vi "UHR-Fleezers Control (host) - 12.0(oscillate_test).vi"() -> ()   [LabVIEW 2014] (continued)
    n3026 = Divide(x=w3808, y=w3807) -> (x/y=→"s/Mean":dbl)
    n3027 = feedback-in #26("Calibration") -> ()
    n3028 = feedback #26(u16 1 ("Calibration")) -> (w3837:u16)
    n3029 = Divide(x="T2 offset_x (mV)", y=1000.0) -> (x/y=w3817:dbl)
    n3030 = case shown="0, Default" "Calibration" {
      tunnel: "T1 a_x (nm/V)" -> [_ w4246 w4267]
      tunnel: "T1 k_x (pN/nm)" -> [_ _ w4257]
      tunnel: "T2 a_x (nm/V)" -> [_ w4245 w4265]
      tunnel: "T2 k_x (pN/nm)" -> [_ _ w4258]
      tunnel: w3818 -> [w4228 w4243 w4263]
      tunnel: w3815 -> [w4227 w4241 w4261]
      tunnel: [w4228 w4240 w4260] -> w3846
      tunnel: [w4227 w4239 w4259] -> w3845
      tunnel: ["T1 X (V)" ("Label.Text") "T1 X (nm)" ("Label.Text") "T1 X (pN)" ("Label.Text")] -> w3834
      tunnel: ["T2 X (V)" ("Label.Text") "T2 X (nm)" ("Label.Text") "T2 X (pN)" ("Label.Text")] -> w3833
      tunnel: ["Position (V)" ("Label.Text") "Position (nm)" ("Label.Text") "Force (pN)" ("Label.Text")] -> w3835
      tunnel: w3817 -> [_ w4231 w4250]
      tunnel: w3819 -> [_ w4234 w4252]
      tunnel: ["Mean (V)" ("Label.Text") "Mean (nm)" ("Label.Text") "Mean (pN)" ("Label.Text")] -> w3830
      tunnel: ["Difference (V)" ("Label.Text") "Difference (nm)" ("Label.Text") "Difference (pN)" ("Label.Text")] -> w3772
      frame 0, Default {
      }
      frame 1 {
        n3031 = Unbundle By Name(w4243) -> ("Y"=w4247:dbl[])
        n3032 = Unbundle By Name(w4241) -> ("Y"=w4232:dbl[])
        n3033 = Subtract(x=w4247, y=w4234) -> (x-y=w4235:dbl[])
        n3034 = Subtract(x=w4232, y=w4231) -> (x-y=w4233:dbl[])
        n3035 = Multiply(x=w4233, y=w4245) -> (x*y=w4242:dbl[])
        n3036 = Multiply(x=w4246, y=w4235) -> (x*y=w4244:dbl[])
        n3037 = Bundle By Name(cluster=w4241, "Y"=w4242) -> (w4239:waveform(dbl))
        n3038 = Bundle By Name(cluster=w4243, "Y"=w4244) -> (w4240:waveform(dbl))
      }
      frame 2 {
        n3039 = Unbundle By Name(w4263) -> ("Y"=w4268:dbl[])
        n3040 = Unbundle By Name(w4261) -> ("Y"=w4266:dbl[])
        n3041 = Subtract(x=w4266, y=w4250) -> (x-y=w4251:dbl[])
        n3042 = Subtract(x=w4268, y=w4252) -> (x-y=w4253:dbl[])
        n3043 = Compound Arithmetic op=MULTIPLY(w4251, w4265, w4258) -> (w4262:dbl[])
        n3044 = Compound Arithmetic op=MULTIPLY(w4257, w4267, w4253) -> (w4264:dbl[])
        n3045 = Bundle By Name(cluster=w4261, "Y"=w4262) -> (w4259:waveform(dbl))
        n3046 = Bundle By Name(cluster=w4263, "Y"=w4264) -> (w4260:waveform(dbl))
      }
    }
    n3047 = Not Equal?(x=w3837, y="Calibration") -> (x != y?=w3798:bool)
    n3048 = case shown="True" w3798 {
      tunnel: w3835 -> [_ w4221]
      tunnel: w3834 -> [_ w4220]
      tunnel: w3833 -> [_ w4219]
      tunnel: w3830 -> [_ w4218]
      tunnel: w3772 -> [_ w4217]
      frame False {
      }
      frame True {
        n3049 = property on="Force" class="WFChart (strict)"("YScale.NameLbl.Text"=w4221) -> ()  [unwired: 2 in, 2 out]
        n3050 = property on="T2 X" class="DigNum (strict)"("Caption.Text"=w4219) -> ()  [unwired: 2 in, 2 out]
        n3051 = property on="T1 X" class="DigNum (strict)"("Caption.Text"=w4220) -> ()  [unwired: 2 in, 2 out]
        n3052 = property on="Mean" class="DigNum (strict)"("Caption.Text"=w4218) -> ()  [unwired: 2 in, 2 out]
        n3053 = property on="Difference" class="DigNum (strict)"("Caption.Text"=w4217) -> ()  [unwired: 2 in, 2 out]
      }
    }
    n3054 = Unbundle By Name(w3818) -> ("Y"=w3821:dbl[])
    n3055 = Unbundle By Name(w3815) -> ("Y"=w3824:dbl[])
    n3056 = Subtract(x=w3821, y=w3819) -> (x-y=w3822:dbl[])
    n3057 = Subtract(x=w3824, y=w3817) -> (x-y=w3823:dbl[])
    n3058 = Multiply(x=w3823, y="T2 a_x (nm/V)") -> (x*y=w3625:dbl[])
    n3059 = Multiply(x="T1 a_x (nm/V)", y=w3822) -> (x*y=w3626:dbl[])
    n3060 = Not(x="Trap Trig. Fl.") -> (.not. x?=w3662:bool)
    n3061 = Multiply(x=w3845, y=-1.0) -> (x*y=w3826:waveform(dbl))
    n3062 = Subtract(x=w3626, y=w3625) -> (x-y=w3814:dbl[])
    n3063 = Unbundle By Name(w3845) -> ("Y"=w3788:dbl[])
    n3064 = Unbundle By Name(w3846) -> ("Y"=w3627:dbl[])
    n3065 = Negate(x=w3814) -> (-x=w3623:dbl[])
    n3066 = Build Array(w3846, w3826) -> (→"Force":waveform(dbl)[])
    n3067 = Subtract(x=w3623, y="Offset (nm)") -> (x-y=w3786:dbl[])
    n3068 = case shown="True" "Read Lateness and Rel Phase" {
      tunnel: w3643 -> [w4192 w4216]
      tunnel: w3642 -> [w4193 w4215]
      tunnel: [w4192 w4214] -> w3812
      tunnel: [w4193 w4213] -> w3811
      frame False {
      }
      frame True {
        n3069 = xnode "Read/Write Control"("FPGA VI Reference In"=w4216, "error in"=w4215) -> ("FPGA VI Reference Out"=w4214:T22, "error out"=w4213:errorcluster, "GI Relative phase"=→"GI relative phase":i16, "Relative phase"=→"Relative phase (AI1)":i16, "AI Late Counter"=→"Late Counter (AI1)":u8, "GI Late Counter"=→"GI Late Counter":u8, "MCL Late Counter"=→"MCL Late Counter":u8, "MCL Relative Phase"=→"Relative Phase (MCL)":i16, "APD Acq Relative Phase"=→"APD Acq Relative Phase":i16, "APD 1 Gate Relative Phase"=→"APD 1 Gate Relative Phase":i16, "APD 2 Gate Relative Phase"=→"APD 2 Gate Relative Phase":i16, "APD Acq Late Counter"=→"APD Acq Late Counter":u8, "APD 1 Gate Late Counter"=→"APD 1 Gate Late Counter":u8, "APD 2 Gate Late Counter"=→"APD 2 Gate Late Counter":u8, "Green FB Relative Phase"=→"Relative phase (Green FB)":i16, "GI Relative phase 2"=→"GI relative phase 2":i16, "GI Late Counter 2"=→"GI Late Counter 2":u8, "Trap Pos FIFO Timeout"=→"Trap Pos FIFO Timeout":u16, "Trap AI FIFO Timeout"=→"Trap AI FIFO Timeout":u16, "RI relative phase"=→"RI relative phase":i16, "RI late counter"=→"RI late counter":u8)
      }
    }
    n3070 = call-poly <vilib>:"Mean.vi"("X"=w3788) -> ("mean"=w3629:dbl)  [unwired: 1 out]
    "T2 X" <- w3629
    n3071 = Negate(x=w3788) -> (-x=w3789:dbl[])
    n3072 = call-poly <vilib>:"Mean.vi"("X"=w3627) -> ("mean"=w3630:dbl)  [unwired: 1 out]
    "T1 X" <- w3630
    n3073 = Negate(x=w3629) -> (-x=w3628:dbl)
    n3074 = Bundle By Name(cluster=w3818, "Y"=w3786) -> (w3763:waveform(dbl))
    "Bead Separation" <- w3763
    n3075 = Add(x=w3627, y=w3789) -> (x+y=w3790:dbl[])
    n3076 = Add(x=w3630, y=w3628) -> (x+y=w3832:dbl)
    n3077 = Subtract(x=w3630, y=w3628) -> (x-y=→"Difference":dbl)
    n3078 = Divide(x=w3790, y=2.0) -> (x/y=→"Vec Mean of T1 T2":dbl[])
    n3079 = Divide(x=w3832, y=2.0) -> (x/y=w3792:dbl)
    "Mean" <- w3792
    n3080 = feedback-in #27("Trap Trig. Fl.") -> ()
    n3081 = feedback #27("Trap Trig. Fl.") -> (w3660:bool)
    n3082 = And(x=w3662, y=w3660) -> (x .and. y?=w3661:bool)
    n3083 = case "If have just turned off triggering" shown="True" w3661 {
      tunnel: w3643 -> [_ w4022]
      tunnel: w3642 -> [_ w4021]
      frame False {
      }
      frame True {
        w4020 = FALSE ("FPGA Trap Trig")
        n3084 = xnode "Read/Write Control"("FPGA VI Reference In"=w4022, "error in"=w4021, "FPGA Trap Trig"=w4020) -> ("FPGA VI Reference Out"=w4019:T22, "error out"=w4018:errorcluster)
        n3085 = xnode "Read/Write Control"("FPGA VI Reference In"=w4019, "error in"=w4018, "TTrig?"=w4020) -> ()  [unwired: 2 out]
        n3086 = local write "Initializing"(FALSE ("Initializing")) -> ()
        n3087 = local write "Triggered"(FALSE ("Triggered")) -> ()
        n3088 = local write "Waiting"(FALSE ("Waiting")) -> ()
      }
    }
    n3089 = Not(x=w3660) -> (.not. x?=w3673:bool)
    n3090 = And(x="Trap Trig. Fl.", y=w3673) -> (x .and. y?=w3670:bool)
    n3091 = local read "Tether"() -> (w3793:bool)
    n3092 = Or(x=w3670, y="Reinitialize") -> (x .or. y?=w3656:bool)
    n3093 = feedback #28(w3666) -> (w3671:string)
    n3094 = Select(t=w3666, s=w3670, f=w3671) -> (s? t:f=w3665:string)
    n3095 = Select(t=w3666, s="Reinitialize", f=w3665) -> (s? t:f=w3664:string)
    n3096 = feedback #29(0) -> (w3668:i32)
    n3097 = feedback #30(w3786) -> (w3785:dbl[])
    n3098 = Build Array (concatenate)(w3786, w3785) -> (w3624:dbl[])
    n3099 = case "For determining if there is a tether still" shown="True" w3793 {
      tunnel: w3792 -> [_ w4146]
      frame False {
      }
      frame True {
        n3100 = Greater?(x="Lost Tether Alarm Threshold (pN)", y=w4146) -> (0:w4144:bool)
        n3101 = case shown="True" w4144 {
          frame False {
          }
          frame True {
            w4147 = TRUE
            w4151 = FALSE ("Multiple tether")
            w4152 = FALSE ("Value (Signaling)")
            n3102 = flat-sequence {
              frame #0 {
                # "stop only if saving"
                n3103 = local read "Saving..."() -> (w4164:bool)
                n3104 = And(x=w4164, y="TA Cancel Save?") -> (x .and. y?=w4163:bool)
                n3105 = local write "Stop Saving"(w4163) -> ()
              }
              frame #1 {
                n3106 = case shown="True" "TA Green Off?" {
                  frame False {
                  }
                  frame True {
                    w4167 = FALSE ("Fl. Triggered...")
                    n3107 = local write "Fl. Triggered..."(w4167) -> ()
                    n3108 = property on="Green ON/Interlacing" class="Bool (strict)"("Val(Sgnl)"=w4167) -> ()  [unwired: 2 in, 2 out]
                  }
                }
              }
            }
            n3109 = local read "Time tether formed"() -> (w4158:timestamp)
            n3110 = Get Date/Time In Seconds() -> (seconds since 1Jan1904=w4159:timestamp)
            n3111 = Subtract(x=w4159, y=w4158) -> (x-y=w4157:dbl)
            n3112 = Number To Decimal String(number=w4157) -> (decimal integer string=w4154:string)  [unwired: 1 out]
            n3113 = local read "Messages"() -> (w4161:string)
            n3114 = call <vilib>:"Beep.vi"("use system alert? (T)"=FALSE, "duration (msec)"=u32 200, "frequency (Hz)"=u32 200) -> ()  [unwired: 9 out]
            n3115 = Concatenate Strings("Lost tether (" ("Message to add"), w4154, " s)." ("string")) -> (w4156:string)
            n3116 = local write "Tether"(FALSE ("Tether")) -> ()
            n3117 = call "Update messages.vi"("Message to add"=w4156, "Old message string"=w4161) -> ("New message string"=w4160:string)
            n3118 = local write "Messages"(w4160) -> ()
            n3119 = local write "Pause dwell"(w4152) -> ()
            n3120 = property on="Fl. Triggered..." class="Bool (strict)"("Val(Sgnl)"=w4152) -> ()  [unwired: 2 in, 2 out]
            n3121 = local write "Dip for Protein"(w4152) -> ()
            n3122 = property on="Trap Pos. FB ON" class="Bool (strict)"("Val(Sgnl)"=w4152) -> ()  [unwired: 2 in, 2 out]
            n3123 = property on="Trap Trig. Fl." class="Bool (strict)"("Val(Sgnl)"=w4152) -> ()  [unwired: 2 in, 2 out]
            n3124 = local write "Multiple tether"(w4151) -> ()
            n3125 = local write "Bad fit"(w4151) -> ()
            n3126 = local write "Hysteresis"(w4151) -> ()
            n3127 = local write "Good tether"(w4151) -> ()
            n3128 = local write "Save scans"(w4147) -> ()
            n3129 = local write "Restart DMA? (AOD)"(w4147) -> ()
          }
        }
      }
    }
    n3130 = case "For triggering actions based on the trap position (e.g., turning the excitation laser on if trap under feedback moves so far)" shown="True" "Trap Trig. Fl." {
      tunnel: w3651 -> [_ w4035]
      tunnel: w3664 -> [_ w4034]
      tunnel: ["" ("t") w4033] -> w3672
      tunnel: w3656 -> [_ w4032]
      tunnel: [0 ("t") w4031] -> w3669
      tunnel: w3668 -> [_ w4030]
      tunnel: w3643 -> [_ w4029]
      tunnel: w3642 -> [_ w4028]
      frame False {
      }
      frame True {
        n3131 = case shown="\"Wait for trigger\"" w4034 {
          tunnel: w4035 -> [w4052 _ _ w4100]
          tunnel: [w4049 w4081 "" ("t") w4103] -> w4033
          tunnel: w4032 -> [_ _ _ w4091]
          tunnel: [w4048 w4078 0 ("t") w4092] -> w4031
          tunnel: w4030 -> [_ w4080 _ w4098]
          tunnel: w4029 -> [w4037 w4075 _ w4094]
          tunnel: w4028 -> [w4036 w4074 _ w4093]
          frame "Wait for trigger" {
            n3132 = local read "Trap Trig. (FPGA)"() -> (w4040:bool)
            n3133 = Subtract(x=w4052, y="Mean T1 Position\nto compare (nm)") -> (x-y=w4045:dbl[])
            n3134 = call <vilib>:"Std Deviation and Variance.vi"("X"=w4045) -> ("mean"=→"mean":dbl, "standard deviation"=→"standard\ndeviation":dbl)  [unwired: 1 in, 1 out]
            n3135 = Array Max & Min(array=w4045) -> (max value=→"max value":dbl, min value=→"min value":dbl)  [unwired: 2 out]
            n3136 = Greater?(x=w4045, y="Threshold (nm)") -> (0:w4055:bool[])
            n3137 = case shown="True" w4040 {
              tunnel: w4037 -> [_ w4061]
              tunnel: w4036 -> [_ w4060]
              tunnel: [FALSE ("TTrig?") w4059] -> w4043
              frame False {
              }
              frame True {
                n3138 = xnode "Read/Write Control"("FPGA VI Reference In"=w4061, "error in"=w4060) -> ("TTrig?"=w4059:bool)  [unwired: 2 out]
              }
            }
            n3139 = Or Array Elements(Boolean array=w4055) -> (logical OR=w4042:bool)
            n3140 = Select(t=w4043, s=w4040, f=w4042) -> (s? t:f=w4041:bool)
            n3141 = Not(x=w4040) -> (.not. x?=w4039:bool)
            n3142 = And(x=w4041, y=w4039) -> (x .and. y?=w4038:bool)
            n3143 = Select(t="Triggered", s=w4041, f="Wait for trigger") -> (s? t:f=w4049:string)
            n3144 = case shown="True" w4041 {
              tunnel: [0 0] -> w4048
              tunnel: w4037 -> [_ w4066]
              tunnel: w4036 -> [_ w4065]
              frame False {
                "Waiting" <- TRUE ("Waiting")
              }
              frame True {
                n3145 = xnode "Read/Write Control"("FPGA VI Reference In"=w4066, "error in"=w4065, "TTrig?"=FALSE) -> ()  [unwired: 2 out]
                n3146 = local read "Messages"() -> (w4069:string)
                n3147 = call <vilib>:"Beep.vi"() -> ()  [unwired: 12 in]
                n3148 = call "Update messages.vi"("Message to add"="Unwinding trigger.", "Old message string"=w4069) -> ("New message string"=w4070:string)
                n3149 = local write "Messages"(w4070) -> ()
                n3150 = local write "Waiting"(FALSE ("Waiting")) -> ()
                "Triggered" <- TRUE ("Triggered")
              }
            }
            n3151 = case "Only need to turn on laser if host triggered" shown="True" w4038 {
              frame False {
              }
              frame True {
                n3152 = property on="Green ON/Interlacing" class="Bool (strict)"("Val(Sgnl)"=TRUE ("Value (Signaling)")) -> ()  [unwired: 2 in, 2 out]
              }
            }
          }
          frame "Triggered" {
            n3153 = local read "Trap Trig. (FPGA)"() -> (w4077:bool)
            n3154 = Increment(x=w4080) -> (x+1=w4078:i32)
            n3155 = Greater Or Equal?(x=w4078, y="Fl. ON time (n)") -> (x >= y?=w4076:bool)
            n3156 = Select(t="Wait for trigger", s=w4076, f="Triggered" ("t")) -> (s? t:f=w4081:string)
            n3157 = And(x=w4076, y=w4077) -> (x .and. y?=w4073:bool)
            n3158 = case shown="True" w4073 {
              tunnel: w4075 -> [_ w4085]
              tunnel: w4074 -> [_ w4084]
              frame False {
              }
              frame True {
                n3159 = xnode "Read/Write Control"("FPGA VI Reference In"=w4085, "error in"=w4084, "FPGA Trap Trig"=TRUE) -> ()  [unwired: 2 out]
              }
            }
            n3160 = case shown="True" w4076 {
              frame False {
              }
              frame True {
                w4087 = FALSE ("Value (Signaling)")
                n3161 = local write "Triggered"(w4087) -> ()
                n3162 = local write "Waiting"(TRUE ("Waiting")) -> ()
                n3163 = property on="Green ON/Interlacing" class="Bool (strict)"("Val(Sgnl)"=w4087) -> ()  [unwired: 2 in, 2 out]
              }
            }
          }
          frame "Do nothing" {
          }
          frame "Initialize", Default {
            n3164 = Increment(x=w4098) -> (x+1=w4102:i32)
            n3165 = Select(t=1, s=w4091, f=w4102) -> (s? t:f=w4092:i32)
            n3166 = feedback #31(w4100) -> (w4106:dbl[])
            n3167 = Build Array (concatenate)(w4100, w4106) -> (w4099:dbl[])
            n3168 = Greater Or Equal?(x=w4092, y="Wait to get offset (n)") -> (x >= y?=w4095:bool)
            n3169 = Select(t=w4100, s=w4091, f=w4099) -> (s? t:f=w4101:dbl[])
            n3170 = feedback-in #31(w4101) -> ()
            n3171 = call-poly <vilib>:"Mean.vi"("X"=w4101) -> ("mean"=w4096:dbl)  [unwired: 1 out]
            n3172 = local write "Mean T1 Position\nto compare (nm)"(w4096) -> ()
            n3173 = case shown="True" w4091 {
              tunnel: w4094 -> [_ w4112]
              tunnel: w4093 -> [_ w4111]
              frame False {
              }
              frame True {
                w4108 = FALSE ("FPGA Trap Trig")
                n3174 = xnode "Read/Write Control"("FPGA VI Reference In"=w4112, "error in"=w4111, "FPGA Trap Trig"=w4108) -> ("FPGA VI Reference Out"=w4110:T22, "error out"=w4109:errorcluster)
                n3175 = xnode "Read/Write Control"("FPGA VI Reference In"=w4110, "error in"=w4109, "TTrig?"=w4108) -> ()  [unwired: 2 out]
              }
            }
            n3176 = Select(t="Wait for trigger", s=w4095, f="Initialize") -> (s? t:f=w4103:string)
            n3177 = case shown="True" w4095 {
              tunnel: w4096 -> [_ w4115]
              tunnel: w4094 -> [_ w4124]
              tunnel: w4093 -> [_ w4123]
              frame False {
                n3178 = local write "Waiting"(FALSE ("Waiting")) -> ()
                "Initializing" <- TRUE ("Initializing")
              }
              frame True {
                n3179 = local read "Threshold (nm)"() -> (w4127:dbl)
                n3180 = local read "AOM X Cal (nm/MHz)"() -> (w4126:dbl)
                n3181 = Add(x=w4115, y=w4127) -> (x+y=w4128:dbl)
                n3182 = Divide(x=w4128, y=w4126) -> (x/y=w4125:dbl)
                n3183 = call "IR AOM freq to word.vi"("Frequency In (MHz)"=w4125) -> ("Frequency Word Out (double)"=w4122:dbl)
                n3184 = local write "Initializing"(FALSE ("Initializing")) -> ()
                n3185 = local write "Waiting"(TRUE ("Waiting")) -> ()
                n3186 = To Quad Integer(1:w4122) -> (0:w4121:i64)
                n3187 = xnode "Read/Write Control"("FPGA VI Reference In"=w4124, "error in"=w4123, "FPGA TTrig Thresh"=w4121) -> ("FPGA VI Reference Out"=w4118:T22, "error out"=w4117:errorcluster)
                n3188 = xnode "Read/Write Control"("FPGA VI Reference In"=w4118, "error in"=w4117, "FPGA Trap Trig"=TRUE) -> ()  [unwired: 2 out]
              }
            }
          }
        }
      }
    }
    n3189 = feedback-in #28(w3672) -> ()
    n3190 = feedback-in #29(w3669) -> ()
    n3191 = Split 1D Array(array=w3624, index=w3686) -> (first subarray=w3782:dbl[])  [unwired: 1 out]
    n3192 = feedback-in #30(w3782) -> ()
    n3193 = call-poly <vilib>:"Mean.vi"("X"=w3782) -> ("mean"=w3781:dbl)  [unwired: 1 out]
    "Bead Mean (nm)" <- w3781
    n3194 = Subtract(x=w3782, y=w3781) -> (x-y=w3780:dbl[])
    n3195 = Square(x=w3780) -> (x^2=w3779:dbl[])
    n3196 = call-poly <vilib>:"Mean.vi"("X"=w3779) -> ("mean"=w3778:dbl)  [unwired: 1 out]
    n3197 = Square Root(x=w3778) -> (sqrt(x)=w3777:dbl)
    n3198 = Multiply(x=10.0, y=w3777) -> (x*y=→"RMS (Å)":dbl)
    n3199 = xnode ("Read/Write Control")("FPGA VI Reference In"=w3812, "error in"=w3811) -> ("FPGA VI Reference Out"=w3654:T22, "error out"=w3653:errorcluster, "AI2 Y Sum Set 1"=w3907:i16, "AI2 Y Sum Set 2"=w3906:i16, "AI1 X Set 1"=w3714:fxp<+/-,16,1>, "AI1 X Set 2"=w3713:fxp<+/-,16,1>, "Trap Pos FB Int Signal"=→"Trap Pos FB Int Signal":fxp<+/-,24,9>, "Trap Pos FB Int-Norm Signal"=→"Trap Pos FB Int-Norm Signal":fxp<+/-,16,1>, "Trap Pos FB Action"=w3707:i64, "Scanning"=→"AOD Scanning":bool, "Scan I"=→"AOD Scan I":u64, "Scanning MCL"=w3909:bool, "Scan I (MCL)"=→"MCL Scan I":u64, "Green FB Sum"=w3849:i16, "Trap Pos FB Action"=w3641:i64, "Wiggling 1"=→"Wiggling T1":bool, "TTrig Fin Thresh"=w3637:i64, "Wiggling 2"=→"Wiggling T2":bool, "Red FB Sum"=w3604:i16)  [unwired: 2 out]
    "MCL Scanning" <- w3909
    "Trap Pos FB Action" <- w3707
    n3200 = local read "FB Trig Integrate"() -> (w3635:u32)
    n3201 = Divide(x=w3849, y=3276.7) -> (x/y=w3603:dbl)
    "Green laser intensity (V)" <- w3603
    n3202 = Divide(x=w3604, y=3276.7) -> (x/y=w3602:dbl)
    "Red laser intensity (V)" <- w3602
    n3203 = Divide(x=w3641, y=w3635) -> (x/y=w3634:dbl)
    "TTrig Sig (Int)" <- w3634
    n3204 = Divide(x=w3637, y=w3635) -> (x/y=w3632:dbl)
    "TTrig Fin Thresh (Int)" <- w3632
    n3205 = local read "AOM X Cal (nm/MHz)"() -> (w3640:dbl)
    n3206 = local read "AI2 (V)"() -> (w3908:cluster{"Set 1":dbl, "Set 2":dbl})
    n3207 = Bundle By Name(cluster=w3908, "Set 1"=w3907, "Set 2"=w3906) -> (w3904:cluster{"Set 1":dbl, "Set 2":dbl})
    n3208 = Divide(x=w3707, y=327.67) -> (x/y=w3619:dbl)
    n3209 = local read "Trap X (AI1)"() -> (w3727:T10)
    n3210 = Bundle(w3603, w3602) -> (→"Excitation laser intensities plot":cluster{dbl, dbl})  [unwired: 1 in]
    n3211 = call "IR AOM word double to freq.vi"("Frequency Word In (double)"=w3632) -> ("Frequency Out (MHz)"=w3631:dbl)
    n3212 = call "IR AOM word double to freq.vi"("Frequency Word In (double)"=w3634) -> ("Frequency Out (MHz)"=w3633:dbl)
    n3213 = Divide(x=w3904, y=3276.7) -> (x/y=w3903:cluster{"Set 1":dbl, "Set 2":dbl})
    n3214 = Multiply(x=w3633, y=w3640) -> (x*y=w3639:dbl)
    "TTrig Sig (nm)" <- w3639
    n3215 = Multiply(x=w3631, y=w3640) -> (x*y=w3638:dbl)
    "TTrig Fin Thresh (nm)" <- w3638
    n3216 = local write "AI2 (V)"(w3903) -> ()
    n3217 = local read "Trap Pos. FB Range"() -> (w3618:T12)
    n3218 = Bundle(cluster=w3727, "Trap 1"=w3714, "Trap 2"=w3713) -> (→"Trap X (AI1)":T10)
    n3219 = Bundle(w3639, w3638) -> (→"TTrig":cluster{dbl, dbl})  [unwired: 1 in]
    n3220 = Unbundle(w3618) -> ("output high"=w3617:fxp<+/-,64,32>)  [unwired: 1 out]
    n3221 = Divide(x=w3619, y=w3617) -> (x/y=→"Action (%)":dbl)
    n3222 = flat-sequence "To save data" {
      tunnel: [w4988] -> w3926
      tunnel: [w4989] -> w3925
      tunnel: w3879 -> [w4961]
      tunnel: w3659 -> [w4986]
      tunnel: ["Save Calibration"] -> w3900
      tunnel: w3897 -> [w4985]
      tunnel: [w4979] -> w3896
      tunnel: [w4976] -> w3895
      tunnel: [w4973] -> w3894
      tunnel: w3878 -> [w4975]
      tunnel: w3796 -> [w4969]
      tunnel: [w4969] -> w3795
      tunnel: ["Start Saving"] -> w3765
      tunnel: [w4963] -> w3699
      tunnel: [w4962] -> w3698
      tunnel: w3926 -> [w5228]
      tunnel: w3925 -> [w5227]
      tunnel: w3700 -> [w5226]
      tunnel: w3900 -> [w5225]
      tunnel: w3896 -> [w5223]
      tunnel: w3895 -> [w5222]
      tunnel: w3894 -> [w5221]
      tunnel: w3774 -> [w5220]
      tunnel: w3805 -> [w5219]
      tunnel: w3795 -> [w5218]
      tunnel: w3765 -> [w5217]
      tunnel: w3763 -> [w5216]
      tunnel: w3741 -> [w5215]
      tunnel: w3699 -> [w5214]
      tunnel: w3698 -> [w5213]
      tunnel: w3697 -> [w5212]
      tunnel: w3620 -> [w5211]
      frame #0 {
        n3223 = Or(x="Save N Sets", y="Start Saving") -> (x .or. y?=w4970:bool)
        n3224 = To Double Precision Float(number=w4985) -> (double precision float=w4980:dbl)
        n3225 = Build Array(w4970, "Save Calibration", w4961, w4975) -> (w4984:bool[])
        n3226 = Compound Arithmetic op=OR("Save Calibration", w4961, w4970, w4975) -> (w4987:bool)
        n3227 = Boolean Array To Number(Boolean array=w4984) -> (number=w4982:u32)
        n3228 = feedback #32(FALSE ("Save APD Data\nwith Trap Data")) -> (w4964:bool)
        n3229 = feedback #33(refnum<k0> refnum) -> (w4990:refnum<file>)
        n3230 = feedback #34(refnum<k0> refnum) -> (w4966:refnum<file>)
        n3231 = feedback #35(FALSE ("Save APD Data\nwith Trap Data")) -> (w4974:bool)
        n3232 = feedback #36(refnum<k0> refnum) -> (w4977:refnum<file>)
        n3233 = feedback #37(0) -> (w4992:i32)
        n3234 = feedback #38() -> (w4981:u32)  [unwired: 1 out]
        n3235 = case shown="True" w4987 {
          tunnel: [w4999 1] -> w4988
          tunnel: w4992 -> [w5001 _]
          tunnel: [w5000 w5019] -> w4989
          tunnel: w4990 -> [w5000 _]
          tunnel: w4986 -> [_ w5039]
          tunnel: w4980 -> [_ w5037]
          tunnel: w4982 -> [_ w5040]
          tunnel: [w4998 w5018] -> w4979
          tunnel: w4981 -> [w4998 _]
          tunnel: [w4997 w5016] -> w4976
          tunnel: w4977 -> [w4997 _]
          tunnel: [w4996 w5015] -> w4973
          tunnel: w4974 -> [w4996 _]
          tunnel: "Start Saving" -> [_ w5013]
          tunnel: w4969 -> [_ w5012]
          tunnel: [w4995 w5003] -> w4962
          tunnel: w4966 -> [w4995 _]
          tunnel: [w4994 w5002] -> w4963
          tunnel: w4964 -> [w4994 _]
          frame False {
            n3236 = Increment(x=w5001) -> (x+1=w4999:i32)
          }
          frame True {
            w5009 = FALSE ("Start Saving")
            w5014 = 9.0  # File Version
            w5022 = FALSE ("prepend array or string size? (T)")
            w5020 = T29."big-endian, network order" ("byte order (0:big-endian, network order)")
            n3237 = local read "BD 1 Frequency 1 (MHz)"() -> (w5036:dbl)
            n3238 = local read "BD 2 Frequency 1 (MHz)"() -> (w5035:dbl)
            n3239 = local read "BD 1 Frequency 2 (MHz)"() -> (w5034:dbl)
            n3240 = local read "BD 2 Frequency 2 (MHz)"() -> (w5033:dbl)
            n3241 = local read "BD 1 Frequency 3 (MHz)"() -> (w5032:dbl)
            n3242 = local read "BD 2 Frequency 3 (MHz)"() -> (w5031:dbl)
            n3243 = Array Size(array=w5012) -> (size(s)=w5011:i32)
            n3244 = To Double Precision Float(number=w5011) -> (double precision float=w5010:dbl)
            n3245 = local write "Save Calibration"(w5009) -> ()
            n3246 = local write "Start Saving"(w5009) -> ()
            n3247 = Build Array("Save APD Data\nwith Trap Data", "Save Trap Pos. Data") -> (w5006:bool[])
            n3248 = Boolean Array To Number(Boolean array=w5006) -> (number=w5005:u32)
            n3249 = Build Array(w5036, w5035, w5034, w5033, w5032, w5031) -> (w5030:dbl[])
            n3250 = case shown="1, Default" w5040 {
              tunnel: w5039 -> [w5113 w5135 w5151 w5189]
              tunnel: w5010 -> [w5118 w5142 w5171 w5208]
              tunnel: w5037 -> [w5117 w5141 w5170 w5207]
              tunnel: [w5114 w5137 w5162 w5199] -> w5028
              tunnel: [w5106 "Cal sets to save" w5152 w5190] -> w5018
              tunnel: w5030 -> [w5115 w5138 w5164 w5201]
              tunnel: "Save APD Data\nwith Trap Data" -> [w5112 _ w5148 w5187]
              tunnel: [w5112 FALSE ("Save APD Data\nwith Trap Data") w5148 w5187] -> w5015
              tunnel: w5014 -> [w5109 w5132 w5146 w5185]
              tunnel: w5013 -> [w5108 _ _ _]
              tunnel: [w5100 "Active cal?" w5145 w5175] -> w5002
              tunnel: "Save Trap Pos. Data" -> [w5100 _ w5145 w5175]
              tunnel: w5005 -> [w5099 _ w5144 w5174]
              frame 1, Default {
                # "timeseries"
                n3251 = case shown="True" "Profile" {
                  tunnel: [w5121 w5125] -> w5104
                  tunnel: [w5121 w5124] -> w5103
                  tunnel: [w5121 w5123] -> w5102
                  tunnel: [w5121 w5122] -> w5101
                  frame False {
                    w5121 = 0.0 ("f")
                  }
                  frame True {
                    n3252 = local read "Current Position"() -> (w5126:cluster{dbl, dbl, dbl})
                    n3253 = local read "Y change (mm)"() -> (w5122:dbl)
                    n3254 = Unbundle(w5126) -> (w5125:dbl, w5124:dbl, w5123:dbl)
                  }
                }
                n3255 = local read "Save ave N"() -> (w5120:dbl)
                n3256 = Multiply(x=w5120, y=w5113) -> (x*y=w5119:dbl)
                n3257 = To Double Precision Float(number=w5099) -> (double precision float=w5111:dbl)
                n3258 = Select(t=4.0, s="Profile", f=0.0) -> (s? t:f=w5095:dbl)
                n3259 = Build Array(w5109, w5113, w5119, w5118, w5117, w5095) -> (w5116:dbl[])
                n3260 = Build Array(w5111, w5104, w5103, w5102, w5101) -> (w5110:dbl[])
                n3261 = Select(t=u32 4000000000, s=w5108, f="N sets to save") -> (s? t:f=w5106:u32)
                n3262 = Build Array (concatenate)(w5116, w5115, w5110) -> (w5114:dbl[])
              }
              frame 2 {
                w5134 = 0.0 ("f")
                # "If doing active calibration,\nalso save trap position file"
                # "calibration"
                n3263 = property on="Wiggle" class="Bool (strict)"("Val(Sgnl)"="Active cal?") -> ()  [unwired: 2 in, 2 out]
                n3264 = Select(t=2.0, s="Active cal?", f=0.0) -> (s? t:f=w5128:dbl)
                n3265 = Build Array(w5128, w5134, w5134, w5134, w5134) -> (w5133:dbl[])
                n3266 = Build Array(w5132, w5135, w5135, w5142, w5141, 1.0 ("t")) -> (w5139:dbl[])
                n3267 = Build Array (concatenate)(w5139, w5138, w5133) -> (w5137:dbl[])
                "Calibrating..." <- TRUE ("Calibrating...")
              }
              frame 4 {
                w5149 = 0.0 ("f")
                # "scan dir (x/y = 0/1)"
                # "cycles/step"
                # "n scans (f/b)"
                # "steps"
                # "freq. range"
                # "AOD raster scan"
                n3268 = local read "Number of F/B Scans (AOD)"() -> (w5156:u16)
                n3269 = local read "Cycles/step (AOD)"() -> (w5158:u64)
                n3270 = local read "Scan Range (MHz)"() -> (w5161:dbl)
                n3271 = local read "Scan steps (AOD)"() -> (w5160:u64)
                n3272 = local read "Scan BD"() -> (w5168:bool)
                n3273 = local read "Save ave N"() -> (w5173:dbl)
                n3274 = Boolean To (0,1)(Boolean=w5168) -> (0, 1=w5167:i16)
                n3275 = To Double Precision Float(number=w5156) -> (double precision float=w5155:dbl)
                n3276 = To Double Precision Float(number=w5160) -> (double precision float=w5159:dbl)
                n3277 = To Double Precision Float(number=w5158) -> (double precision float=w5157:dbl)
                n3278 = To Double Precision Float(number=w5167) -> (double precision float=w5166:dbl)
                n3279 = Multiply(x=w5173, y=w5151) -> (x*y=w5172:dbl)
                n3280 = To Double Precision Float(number=w5144) -> (double precision float=w5150:dbl)
                n3281 = Build Array(w5150, w5149, w5149, w5149, w5149) -> (w5147:dbl[])
                n3282 = local read "N sets should be saved"() -> (w5153:dbl)
                n3283 = Build Array(w5166, w5161, w5159, w5157, w5155) -> (w5163:dbl[])
                n3284 = Build Array(w5146, w5151, w5172, w5171, w5170, 2.0 ("t")) -> (w5165:dbl[])
                n3285 = Round Toward +Infinity(x=w5153) -> (ceil(x): smallest int >= x=w5154:dbl)
                n3286 = Build Array (concatenate)(w5165, w5164, w5147, w5163) -> (w5162:dbl[])
                n3287 = To Unsigned Long Integer(number=w5154) -> (unsigned 32bit integer=w5152:u32)
              }
              frame 8 {
                w5182 = 0.0 ("f")
                # "MCL raster scan"
                n3288 = local read "Number of scans (MCL)"() -> (w5177:u64)
                n3289 = local read "Scan lines (y)"() -> (w5176:u64)
                n3290 = local read "2D or 1D Scan"() -> (w5179:bool)
                n3291 = local read "Scan Range (V)\n(of steps)"() -> (w5198:dbl)
                n3292 = local read "Fast Scan Dir"() -> (w5205:bool)
                n3293 = local read "Cycles/step (MCL)"() -> (w5195:u64)
                n3294 = local read "Scan steps (MCL)"() -> (w5197:u64)
                n3295 = Select(t=w5176, s=w5179, f=w5177) -> (s? t:f=w5178:u64)
                n3296 = Boolean To (0,1)(Boolean=w5179) -> (0, 1=w5181:i16)
                n3297 = local read "Save ave N"() -> (w5210:dbl)
                n3298 = local read "Initial X"() -> (w5184:dbl)
                n3299 = local read "Initial Y"() -> (w5183:dbl)
                n3300 = To Double Precision Float(number=w5181) -> (double precision float=w5180:dbl)
                n3301 = Boolean To (0,1)(Boolean=w5205) -> (0, 1=w5204:i16)
                n3302 = To Double Precision Float(number=w5178) -> (double precision float=w5193:dbl)
                n3303 = To Double Precision Float(number=w5197) -> (double precision float=w5196:dbl)
                n3304 = To Double Precision Float(number=w5195) -> (double precision float=w5194:dbl)
                n3305 = To Double Precision Float(number=w5204) -> (double precision float=w5203:dbl)
                n3306 = Multiply(x=w5210, y=w5189) -> (x*y=w5209:dbl)
                n3307 = To Double Precision Float(number=w5174) -> (double precision float=w5188:dbl)
                n3308 = local read "N sets should be saved (MCL)"() -> (w5191:dbl)
                n3309 = Build Array(w5188, w5180, w5182, w5182, w5182) -> (w5186:dbl[])
                n3310 = Build Array(w5203, w5198, w5196, w5194, w5193, w5184, w5183) -> (w5200:dbl[])
                n3311 = Build Array(w5185, w5189, w5209, w5208, w5207, 3.0 ("t")) -> (w5202:dbl[])
                n3312 = Round Toward +Infinity(x=w5191) -> (ceil(x): smallest int >= x=w5192:dbl)
                n3313 = Build Array (concatenate)(w5202, w5201, w5186, w5200) -> (w5199:dbl[])
                n3314 = To Unsigned Long Integer(number=w5192) -> (unsigned 32bit integer=w5190:u32)
              }
            }
            n3315 = local read "Index"() -> (w5045:dbl)
            n3316 = call "Create new save file.vi"("Insert"="", "Ext"=".dat", "Index In"=w5045) -> ("Path Out"=w5004:path, "Index Out"=w5017:dbl)
            n3317 = local write "Save file name"(w5004) -> ()
            n3318 = local write "Index"(w5017) -> ()
            n3319 = local write "Save index"(w5017) -> ()
            n3320 = Array Size(array=w5028) -> (size(s)=w5029:i32)
            n3321 = Open/Create/Replace File(file path (use dialog)=w5004, operation (0:open)=T30."create", access (0:read/write)=enum16{"read/write", "read-only", "write-only"}."write-only") -> (refnum out=w5042:refnum<file>)  [unwired: 1 in, 4 out]
            n3322 = local write "Saving..."(TRUE ("Saving...")) -> ()
            n3323 = To Double Precision Float(number=w5029) -> (double precision float=w5027:dbl)
            n3324 = String Length(string="Comment (data description)") -> (length=w5025:i32)
            n3325 = To Double Precision Float(number=w5025) -> (double precision float=w5024:dbl)
            n3326 = Deny Access(7:w5042) -> (3:w5041:refnum<file>)  [unwired: 1 in, 2 out]
            n3327 = Build Array (concatenate)(w5027, w5028, w5024) -> (w5026:dbl[])
            n3328 = case "If fluorescence data to be saved" shown="True" w5015 {
              tunnel: w5004 -> [_ w5094]
              tunnel: [refnum<k0> refnum w5074] -> w5016
              frame False {
              }
              frame True {
                w5073 = 0.0
                n3329 = local read "APD Integration Time (s)"() -> (w5079:dbl)
                n3330 = local read "N APD Samp/step"() -> (w5072:dbl)
                n3331 = Path To String(path=w5094) -> (string=w5093:string)
                n3332 = String Length(string=w5093) -> (length=w5092:i32)
                n3333 = Subtract(x=w5092, y=4) -> (x-y=w5090:i32)
                n3334 = String Subset(string=w5093, length (rest)=w5090) -> (substring=w5089:string)  [unwired: 1 out]
                n3335 = Build Array(w5079, w5072, w5073, w5073, w5073, w5073, w5073, w5073) -> (w5076:dbl[])
                n3336 = Concatenate Strings(w5089, "_fl.dat" ("string")) -> (w5087:string)
                n3337 = Array Size(array=w5076) -> (size(s)=w5078:i32)
                n3338 = String To Path(string=w5087) -> (path=w5083:path)
                n3339 = Open/Create/Replace File(file path (use dialog)=w5083, operation (0:open)=T30."create", access (0:read/write)=enum16{"read/write", "read-only", "write-only"}."write-only") -> (refnum out=w5084:refnum<file>)  [unwired: 1 in, 4 out]
                n3340 = Deny Access(7:w5084) -> (3:w5080:refnum<file>)  [unwired: 1 in, 2 out]
                n3341 = To Double Precision Float(number=w5078) -> (double precision float=w5077:dbl)
                n3342 = Build Array (concatenate)(w5077, w5076) -> (w5075:dbl[])
                n3343 = Write to Binary File(file (use dialog)=w5080, data=w5075, 5:FALSE ("prepend array or string size? (T)"), 9:T29."big-endian, network order" ("byte order (0:big-endian, network order)")) -> (refnum out=w5074:refnum<file>)  [unwired: 1 in, 3 out]
              }
            }
            n3344 = case shown="True" w5002 {
              tunnel: w5004 -> [_ w5056]
              tunnel: [refnum<k0> refnum w5055] -> w5003
              frame False {
              }
              frame True {
                w5051 = 0.0 ("element")
                n3345 = Path To String(path=w5056) -> (string=w5070:string)
                n3346 = Build Array(w5051, w5051, w5051, w5051, w5051, w5051, w5051, w5051) -> (w5052:dbl[])
                n3347 = String Length(string=w5070) -> (length=w5069:i32)
                n3348 = Subtract(x=w5069, y=4) -> (x-y=w5067:i32)
                n3349 = Array Size(array=w5052) -> (size(s)=w5054:i32)
                n3350 = String Subset(string=w5070, length (rest)=w5067) -> (substring=w5066:string)  [unwired: 1 out]
                n3351 = To Double Precision Float(number=w5054) -> (double precision float=w5053:dbl)
                n3352 = Concatenate Strings(w5066, "_pos.dat" ("string")) -> (w5064:string)
                n3353 = Build Array (concatenate)(w5053, w5052) -> (w5050:dbl[])
                n3354 = String To Path(string=w5064) -> (path=w5060:path)
                n3355 = Open/Create/Replace File(file path (use dialog)=w5060, operation (0:open)=T30."create", access (0:read/write)=enum16{"read/write", "read-only", "write-only"}."write-only") -> (refnum out=w5061:refnum<file>)  [unwired: 1 in, 4 out]
                n3356 = Deny Access(7:w5061) -> (3:w5057:refnum<file>)  [unwired: 1 in, 2 out]
                n3357 = Write to Binary File(file (use dialog)=w5057, data=w5050, 5:FALSE ("prepend array or string size? (T)"), 9:T29."big-endian, network order" ("byte order (0:big-endian, network order)")) -> (refnum out=w5055:refnum<file>)  [unwired: 1 in, 3 out]
              }
            }
            n3358 = Write to Binary File(file (use dialog)=w5041, data=w5026, 5:w5022, 9:w5020) -> (refnum out=w5023:refnum<file>)  [unwired: 1 in, 3 out]
            n3359 = Write to Binary File(file (use dialog)=w5023, data="Comment (data description)", 5:w5022, 9:w5020) -> (refnum out=w5019:refnum<file>)  [unwired: 1 in, 3 out]
          }
        }
        n3360 = feedback-in #32(w4963) -> ()
        n3361 = feedback-in #33(w4989) -> ()
        n3362 = feedback-in #34(w4962) -> ()
        n3363 = feedback-in #35(w4973) -> ()
        n3364 = feedback-in #36(w4976) -> ()
        n3365 = feedback-in #37(w4988) -> ()
        n3366 = feedback-in #38(w4979) -> ()
      }
      frame #1 {
        n3367 = local read "Saving..."() -> (w5224:bool)
        n3368 = case shown="True" w5224 {
          tunnel: w5228 -> [_ w5240]
          tunnel: w5227 -> [_ w5253]
          tunnel: w5226 -> [_ w5249]
          tunnel: w5225 -> [_ w5248]
          tunnel: w5223 -> [_ w5229]
          tunnel: w5222 -> [_ w5243]
          tunnel: w5221 -> [_ w5242]
          tunnel: w5220 -> [_ w5241]
          tunnel: w5219 -> [_ w5239]
          tunnel: w5218 -> [_ w5237]
          tunnel: w5217 -> [_ w5236]
          tunnel: w5216 -> [_ w5235]
          tunnel: w5215 -> [_ w5234]
          tunnel: w5214 -> [_ w5233]
          tunnel: w5213 -> [_ w5232]
          tunnel: w5212 -> [_ w5231]
          tunnel: w5211 -> [_ w5230]
          frame False {
          }
          frame True {
            n3369 = Multiply(x=w5240, y=w5239) -> (x*y=→"Time (s)":dbl)
            n3370 = Less Or Equal?(x=w5240, y=w5229) -> (x <= y?=w5251:bool)
            n3371 = Or(x="Stop Saving", y="Abort save 2") -> (x .or. y?=w5244:bool)
            n3372 = Not(x=w5244) -> (.not. x?=w5252:bool)
            n3373 = And(x=w5251, y=w5252) -> (x .and. y?=w5250:bool)
            n3374 = case shown="True" w5250 {
              tunnel: w5253 -> [w5261 w5336]
              tunnel: [0.0 w5339] -> w5247
              tunnel: w5240 -> [_ w5337]
              tunnel: w5229 -> [_ w5338]
              tunnel: w5249 -> [_ w5333]
              tunnel: w5248 -> [_ _]
              tunnel: w5243 -> [w5259 w5326]
              tunnel: w5242 -> [w5258 w5327]
              tunnel: w5241 -> [_ w5325]
              tunnel: w5237 -> [_ w5324]
              tunnel: w5236 -> [_ w5268]
              tunnel: w5235 -> [_ w5317]
              tunnel: w5234 -> [_ w5295]
              tunnel: w5233 -> [w5255 w5277]
              tunnel: w5232 -> [w5256 w5276]
              tunnel: w5231 -> [_ w5273]
              tunnel: w5230 -> [_ w5271]
              frame False {
                w5257 = FALSE
                n3375 = Close File(refnum=w5261) -> ()  [unwired: 1 in, 2 out]
                n3376 = case shown="True" w5258 {
                  tunnel: w5259 -> [_ w5263]
                  frame False {
                  }
                  frame True {
                    n3377 = Close File(refnum=w5263) -> ()  [unwired: 1 in, 2 out]
                  }
                }
                n3378 = case shown="True" w5255 {
                  tunnel: w5256 -> [_ w5262]
                  frame False {
                  }
                  frame True {
                    n3379 = Close File(refnum=w5262) -> ()  [unwired: 1 in, 2 out]
                  }
                }
                n3380 = call <vilib>:"Beep.vi"() -> ()  [unwired: 3 in, 9 out]
                n3381 = local write "Raster Scanning..."(w5257) -> ()
                n3382 = local write "Calibrating..."(w5257) -> ()
                n3383 = property on="Abort wiggle" class="Bool (strict)"("Val(Sgnl)"=TRUE) -> ()  [unwired: 2 in, 2 out]
                n3384 = local write "Stop Saving"(w5257) -> ()
                "Saving..." <- w5257
              }
              frame True {
                n3385 = local read "Calibrating..."() -> (w5328:bool)
                n3386 = case "Write fl. data" shown="True" w5327 {
                  tunnel: w5326 -> [_ w5362]
                  tunnel: w5325 -> [_ w5361]
                  frame False {
                  }
                  frame True {
                    n3387 = Write to Binary File(file (use dialog)=w5362, data=w5361, 5:FALSE ("prepend array or string size? (T)"), 9:T29."big-endian, network order" ("byte order (0:big-endian, network order)")) -> ()  [unwired: 1 in, 4 out]
                  }
                }
                n3388 = Greater?(x="Save ave N", y=1.0) -> (0:w5331:bool)
                n3389 = Not(x=w5328) -> (.not. x?=w5330:bool)
                n3390 = And(x=w5330, y=w5331) -> (x .and. y?=w5274:bool)
                n3391 = case shown="True" w5274 {
                  tunnel: w5273 -> [w5342 w5353]
                  tunnel: [w5342 w5345] -> w5272
                  tunnel: "Save ave N" -> [_ w5346]
                  frame False {
                  }
                  frame True {
                    w5343 = 2 ("dimension size")
                    n3392 = Array Size(array=w5353) -> (size(s)=w5347:i32)
                    n3393 = Divide(x=w5347, y=w5343) -> (x/y=w5351:dbl)
                    n3394 = Reshape Array(w5353, w5351, w5343) -> (w5352:u64[][])
                    n3395 = Transpose 2D Array(2D array=w5352) -> (transposed array=w5350:u64[][])
                    n3396 = for {
                      tunnel: w5350 -> [w5355] mode=indexing
                      tunnel: [w5354] -> w5344 mode=indexing
                      tunnel: w5346 -> [w5356]
                      workers-P: _ -> [_]
                      n3397 = call "downsample 1D array - U64.vi"("Ave N"=w5356, "Array In"=w5355) -> ("Array Out"=w5354:u64[])  [unwired: 1 in]
                    }
                    n3398 = Transpose 2D Array(2D array=w5344) -> (transposed array=w5349:u64[][])
                    n3399 = Divide(x=w5347, y=w5346) -> (x/y=w5348:dbl)
                    n3400 = Reshape Array(w5349, w5348) -> (w5345:u64[])
                  }
                }
                n3401 = case shown="True" w5274 {
                  tunnel: w5333 -> [w5365 w5377]
                  tunnel: [w5365 w5369] -> w5329
                  tunnel: "Save ave N" -> [_ w5370]
                  tunnel: w5324 -> [_ w5368]
                  frame False {
                  }
                  frame True {
                    n3402 = Array Size(array=w5377) -> (size(s)=w5371:i32)
                    n3403 = Array Size(array=w5368) -> (size(s)=w5367:i32)
                    n3404 = Divide(x=w5371, y=w5367) -> (x/y=w5375:dbl)
                    n3405 = Reshape Array(w5377, w5375, w5367) -> (w5376:i16[][])
                    n3406 = Transpose 2D Array(2D array=w5376) -> (transposed array=w5374:i16[][])
                    n3407 = for {
                      tunnel: w5374 -> [w5380] mode=indexing
                      tunnel: [w5379] -> w5366 mode=indexing
                      tunnel: w5370 -> [w5378]
                      workers-P: _ -> [_]
                      n3408 = call "downsample 1D array - I16.vi"("Ave N"=w5378, "Array In"=w5380) -> ("Array Out"=w5379:i16[])  [unwired: 1 out]
                    }
                    n3409 = Transpose 2D Array(2D array=w5366) -> (transposed array=w5373:i16[][])
                    n3410 = Divide(x=w5371, y=w5370) -> (x/y=w5372:dbl)
                    n3411 = Reshape Array(w5373, w5372) -> (w5369:i16[])
                  }
                }
                n3412 = Index Array(array=w5295, index=1) -> (element=w5298:waveform(dbl))
                n3413 = Index Array(array=w5295, index=0) -> (element=w5300:waveform(dbl))
                n3414 = Unbundle By Name(w5298) -> ("Y"=w5302:dbl[])
                n3415 = Unbundle By Name(w5300) -> ("Y"=w5310:dbl[])
                n3416 = case "Write trap pos. data" shown="True" w5277 {
                  tunnel: w5276 -> [_ w5358]
                  tunnel: w5272 -> [_ w5357]
                  frame False {
                  }
                  frame True {
                    n3417 = Write to Binary File(file (use dialog)=w5358, data=w5357, 5:FALSE ("prepend array or string size? (T)"), 9:T29."big-endian, network order" ("byte order (0:big-endian, network order)")) -> ()  [unwired: 1 in, 4 out]
                  }
                }
                n3418 = Write to Binary File(file (use dialog)=w5336, data=w5329, 5:FALSE ("prepend array or string size? (T)"), 9:T29."big-endian, network order" ("byte order (0:big-endian, network order)")) -> ()  [unwired: 1 in, 4 out]
                n3419 = feedback #39(w5302) -> (w5304:dbl[])
                n3420 = Build Array (concatenate)(w5304, w5302) -> (w5303:dbl[])
                n3421 = Select(t=w5302, s=w5268, f=w5303) -> (s? t:f=w5288:dbl[])
                n3422 = feedback-in #39(w5288) -> ()
                n3423 = feedback #40(w5310) -> (w5323:dbl[])
                n3424 = Build Array (concatenate)(w5323, w5310) -> (w5322:dbl[])
                n3425 = Select(t=w5310, s=w5268, f=w5322) -> (s? t:f=w5297:dbl[])
                n3426 = feedback-in #40(w5297) -> ()
                n3427 = Divide(x=w5337, y=w5338) -> (x/y=w5340:dbl)
                n3428 = Multiply(x=w5340, y=100.0) -> (x*y=w5339:dbl)
                n3429 = Build Array(w5297, w5288) -> (→"Saved APD":dbl[][])
                n3430 = Array Size(array=w5297) -> (size(s)=w5315:i32)
                n3431 = Unbundle By Name(w5317) -> ("Y"=w5321:dbl[])
                n3432 = Subtract(x=w5315, y="N pts to average") -> (x-y=w5291:i32)
                n3433 = Multiply(x="N pts to average", y=u16 2) -> (x*y=w5292:u16)
                n3434 = Subtract(x=w5315, y=w5292) -> (x-y=w5290:i32)
                n3435 = feedback #41(w5321) -> (w5320:dbl[])
                n3436 = Build Array (concatenate)(w5320, w5321) -> (w5319:dbl[])
                n3437 = Select(t=w5321, s=w5268, f=w5319) -> (s? t:f=w5318:dbl[])
                "Trap Delta Graph" <- w5318
                n3438 = feedback-in #41(w5318) -> ()
                n3439 = Array Subset(array=w5297, index=w5291, length="N pts to average") -> (w5314:dbl[])
                n3440 = Array Subset(array=w5297, index=w5290, length="N pts to average") -> (w5313:dbl[])
                n3441 = Array Subset(array=w5288, index=w5291, length="N pts to average") -> (w5294:dbl[])
                n3442 = Array Subset(array=w5288, index=w5290, length="N pts to average") -> (w5293:dbl[])
                n3443 = Index Array(array=w5271, index=0) -> (element=w5269:waveform(dbl))
                n3444 = call-poly <vilib>:"Mean.vi"("X"=w5314) -> ("mean"=w5312:dbl)  [unwired: 1 out]
                n3445 = call-poly <vilib>:"Mean.vi"("X"=w5294) -> ("mean"=w5287:dbl)  [unwired: 1 out]
                n3446 = call-poly <vilib>:"Mean.vi"("X"=w5313) -> ("mean"=w5311:dbl)  [unwired: 1 out]
                n3447 = call-poly <vilib>:"Mean.vi"("X"=w5293) -> ("mean"=w5286:dbl)  [unwired: 1 out]
                n3448 = Unbundle By Name(w5269) -> ("Y"=w5266:dbl[])
                n3449 = Subtract(x=w5287, y=w5286) -> (x-y=w5278:dbl)
                "Delta Fl. 2" <- w5278
                n3450 = Subtract(x=w5312, y=w5311) -> (x-y=w5309:dbl)
                "Delta Fl. 1" <- w5309
                n3451 = Initialize Array(w5309, 1 ("dimension size")) -> (w5306:dbl[])
                n3452 = Initialize Array(w5278, 1 ("dimension size")) -> (w5283:dbl[])
                n3453 = feedback #42(w5306) -> (w5307:dbl[])
                n3454 = Build Array (concatenate)(w5307, w5306) -> (w5305:dbl[])
                n3455 = feedback #43(w5283) -> (w5284:dbl[])
                n3456 = Build Array (concatenate)(w5284, w5283) -> (w5282:dbl[])
                n3457 = feedback #44(w5266) -> (w5265:dbl[])
                n3458 = Build Array (concatenate)(w5265, w5266) -> (w5267:dbl[])
                n3459 = Select(t=w5266, s=w5268, f=w5267) -> (s? t:f=w5264:dbl[])
                "Saved trap pos" <- w5264
                n3460 = feedback-in #44(w5264) -> ()
                n3461 = Select(t=w5306, s=w5268, f=w5305) -> (s? t:f=w5281:dbl[])
                n3462 = feedback-in #42(w5281) -> ()
                n3463 = Select(t=w5283, s=w5268, f=w5282) -> (s? t:f=w5280:dbl[])
                n3464 = feedback-in #43(w5280) -> ()
                n3465 = Build Array(w5281, w5280) -> (→"Save APD Deriv":dbl[][])
              }
            }
            "Progress" <- w5247
            "Progress 2" <- w5247
          }
        }
      }
    }
    n3466 = local read "wait to reset values"() -> (w3911:bool)
    n3467 = Not(x=w3909) -> (.not. x?=w3912:bool)
    n3468 = And(x=w3912, y=w3911) -> (x .and. y?=w3913:bool)
    n3469 = case "Part of MCL raster scanning: returns to initial positions after scan done" shown="True" w3913 {
      tunnel: w3654 -> [w4782 w4789]
      tunnel: [w4782 w4788] -> w3915
      tunnel: w3653 -> [w4781 w4787]
      tunnel: [w4781 w4786] -> w3910
      frame False {
      }
      frame True {
        w4797 = 10.0 ("y")
        w4796 = 32767.0 ("y")
        # "to return scan values\nafter a synchronous \nAOM scan"
        n3470 = local read "AO2"() -> (w4790:dbl)
        n3471 = local read "AO1"() -> (w4791:dbl)
        n3472 = local write "wait to reset values"(FALSE ("wait to reset values")) -> ()
        n3473 = Multiply(x=w4791, y=w4796) -> (x*y=w4793:dbl)
        n3474 = Multiply(x=w4790, y=w4796) -> (x*y=w4795:dbl)
        n3475 = Divide(x=w4793, y=w4797) -> (x/y=w4792:dbl)
        n3476 = Divide(x=w4795, y=w4797) -> (x/y=w4794:dbl)
        n3477 = To Word Integer(number=w4792) -> (16bit integer=w4798:i16)
        n3478 = To Word Integer(number=w4794) -> (16bit integer=w4799:i16)
        n3479 = local read "Total Counts (ticks)"() -> (w4783:u32)
        n3480 = xnode "Read/Write Control"("FPGA VI Reference In"=w4789, "error in"=w4787, "AO1"=w4798, "AO2"=w4799, "MCL count"=w4783) -> ("FPGA VI Reference Out"=w4788:T22, "error out"=w4786:errorcluster)
        n3481 = local read "Scan Range (V)\n(of steps)"() -> (w4784:dbl)
        n3482 = property on="Scan Range (V)\n(of steps)" class="DigNum (strict)"("Val(Sgnl)"=w4784) -> ()  [unwired: 2 in, 2 out]
      }
    }
    n3483 = node-c288() -> ()  [unwired: 2 out]
  }
  n3484 = VISA Close(VISA resource name=w129, error in (no error)=w128) -> (error out=w172:errorcluster)
  n3485 = call <vilib>:"Simple Error Handler.vi"("error in (no error)"=w172) -> ()  [unwired: 1 in, 8 out]
  n3486 = node-c288(w134) -> ()  [unwired: 1 out]
  n3487 = node-c288(w216) -> ()  [unwired: 1 out]
  n3488 = flat-sequence {
    tunnel: w307 -> [w5384]
    tunnel: w309 -> [w5385]
    tunnel: [w5383] -> w289
    tunnel: [w5382] -> w288
    tunnel: w272 -> [_]
    tunnel: w224 -> [_]
    tunnel: w140 -> [_]
    tunnel: w289 -> [w5386]
    tunnel: w288 -> [w5387]
    frame #0 {
      w5381 = FALSE ("AI to FIFO")
      n3489 = xnode "Read/Write Control"("FPGA VI Reference In"=w5385, "error in"=w5384, "AI to FIFO"=w5381, "APD to FIFO"=w5381) -> ("FPGA VI Reference Out"=w5383:T22, "error out"=w5382:errorcluster)
    }
    frame #1 {
      n3490 = xnode "Close FPGA VI Reference"("FPGA VI Reference In"=w5386, "error in"=w5387) -> ("error out"=→"error out":errorcluster)
    }
  }
